vi "CRYO_MASTER_FULL_RUN2.vi"() -> ()   [LabVIEW 2017] (continued)
          }
          frame #47 {
            n631 = Search 1D Array(1D array=w1178, element=T14."TTH4" ("SensorLocations")) -> (index of element=w1175:i32)  [unwired: 1 in]
            n632 = Index Array(array=w1176, index=w1175) -> (element=→"TTH4":dbl)
          }
          frame #48 {
            n633 = Search 1D Array(1D array=w1183, element="SensorLocation 1") -> (index of element=w1180:i32)  [unwired: 1 in]
            n634 = Index Array(array=w1181, index=w1180) -> (element=→"Temperature 1":dbl)
          }
          frame #49 {
            n635 = Search 1D Array(1D array=w1188, element="SensorLocation 2") -> (index of element=w1185:i32)  [unwired: 1 in]
            n636 = Index Array(array=w1186, index=w1185) -> (element=→"Temperature 2":dbl)
          }
        }
      }
      frame #1 {
        n637 = stacked-sequence {
          tunnel: w1190 -> [w1195 w1200 w1205 w1210 w1215 w1220 w1225 w1230 w1235 w1240 w1245 w1250 w1255 w1260 w1265 w1270 w1275 w1280 w1285]
          tunnel: w1189 -> [w1192 w1198 w1204 w1209 w1214 w1218 w1223 w1228 w1233 w1238 w1243 w1248 w1252 w1257 w1262 w1267 w1272 w1277 w1282]
          frame #0 {
            n638 = Search 1D Array(1D array=w1195, element="Insulation vacuum") -> (index of element=w1193:i32)  [unwired: 1 in]
            n639 = Index Array(array=w1192, index=w1193) -> (element=→"P_ins" →"P (insulation)":dbl)
          }
          frame #1 {
            n640 = Search 1D Array(1D array=w1200, element="4K reservoir pressure") -> (index of element=w1197:i32)  [unwired: 1 in]
            n641 = Index Array(array=w1198, index=w1197) -> (element=→"P_4Kres" →"P (4K reservoir)":dbl)
          }
          frame #2 {
            n642 = Search 1D Array(1D array=w1205, element="3He inlet pressure") -> (index of element=w1203:i32)  [unwired: 1 in]
            n643 = Index Array(array=w1204, index=w1203) -> (element=→"P_3HeIN" →"P (3He IN)":dbl)
          }
          frame #3 {
            n644 = Search 1D Array(1D array=w1210, element="Shield return press.") -> (index of element=w1208:i32)  [unwired: 1 in]
            n645 = Index Array(array=w1209, index=w1208) -> (element=→"P_SldRTN" →"P (shield return)":dbl)
          }
          frame #4 {
            n646 = Search 1D Array(1D array=w1215, element="3He pot pressure") -> (index of element=w1213:i32)  [unwired: 1 in]
            n647 = Index Array(array=w1214, index=w1213) -> (element=→"P_3Hepot" →"P (3He pot)":dbl)
          }
          frame #5 {
            n648 = Search 1D Array(1D array=w1220, element="1Kpot pressure") -> (index of element=w1217:i32)  [unwired: 1 in]
            n649 = Index Array(array=w1218, index=w1217) -> (element=→"P_1Kpot" →"P (1K pot)":dbl)
          }
          frame #6 {
            n650 = Search 1D Array(1D array=w1225, element="Dewar pressure") -> (index of element=w1222:i32)  [unwired: 1 in]
            n651 = Index Array(array=w1223, index=w1222) -> (element=→"P_Dewar" →"P (Dewar)":dbl)
          }
          frame #7 {
            n652 = Search 1D Array(1D array=w1230, element="HEX7 out pressure") -> (index of element=w1227:i32)  [unwired: 1 in]
            n653 = Index Array(array=w1228, index=w1227) -> (element=→"P_HEX7OUT" →"P (HEX7 out)":dbl)
          }
          frame #8 {
            n654 = Search 1D Array(1D array=w1235, element="Diff pressure HEX4") -> (index of element=w1232:i32)  [unwired: 1 in]
            n655 = Index Array(array=w1233, index=w1232) -> (element=→"DP_HEX4" →"DP HEX4":dbl)
          }
          frame #9 {
            n656 = Search 1D Array(1D array=w1240, element="Diff pressure HEX5") -> (index of element=w1237:i32)  [unwired: 1 in]
            n657 = Index Array(array=w1238, index=w1237) -> (element=→"DP_HEX5" →"DP HEX5":dbl)
          }
          frame #10 {
            n658 = Search 1D Array(1D array=w1245, element="1K pump exhaust flow") -> (index of element=w1242:i32)  [unwired: 1 in]
            n659 = Index Array(array=w1243, index=w1242) -> (element=→"F_1" →"F1 (1K pump exhaust) flow":dbl)
          }
          frame #11 {
            n660 = Search 1D Array(1D array=w1250, element="Shield flow") -> (index of element=w1247:i32)  [unwired: 1 in]
            n661 = Index Array(array=w1248, index=w1247) -> (element=→"F_2" →"F2 (shield flow)":dbl)
          }
          frame #12 {
            n662 = Search 1D Array(1D array=w1255, element="4He return flow from HEX7") -> (index of element=w1253:i32)  [unwired: 1 in]
            n663 = Index Array(array=w1252, index=w1253) -> (element=→"F_3" →"F3 (4He rtn flw via HEX7)":dbl)
          }
          frame #13 {
            n664 = Search 1D Array(1D array=w1260, element="3He incoming flow into HEX7") -> (index of element=w1258:i32)  [unwired: 1 in]
            n665 = Index Array(array=w1257, index=w1258) -> (element=→"F_4" →"F4 (3He in to HEX7)":dbl)
          }
          frame #14 {
            n666 = Search 1D Array(1D array=w1265, element="3He pump exhaust flow") -> (index of element=w1263:i32)  [unwired: 1 in]
            n667 = Index Array(array=w1262, index=w1263) -> (element=→"F_5" →"F5 (3He pump ex.)":dbl)
          }
          frame #15 {
            n668 = Search 1D Array(1D array=w1270, element="4K reservoir level") -> (index of element=w1268:i32)  [unwired: 1 in]
            n669 = Index Array(array=w1267, index=w1268) -> (element=→"L3" →"He level (4K)":dbl)
          }
          frame #16 {
            n670 = Search 1D Array(1D array=w1275, element="1K pot level") -> (index of element=w1273:i32)  [unwired: 1 in]
            n671 = Index Array(array=w1272, index=w1273) -> (element=→"L(1K) (a1)" →"He level (1K)":dbl)
          }
          frame #17 {
            n672 = Search 1D Array(1D array=w1280, element="1K pot (b)") -> (index of element=w1278:i32)  [unwired: 1 in]
            n673 = Index Array(array=w1277, index=w1278) -> (element=→"1K pot(b1)" →"He level (1K) b":dbl)
          }
          frame #18 {
            n674 = Search 1D Array(1D array=w1285, element="3He pot") -> (index of element=w1283:i32)  [unwired: 1 in]
            n675 = Index Array(array=w1282, index=w1283) -> (element=→"3He pot level" →"He level (3He)":dbl)
          }
        }
      }
    }
    n676 = case shown="False" w830 {
      tunnel: [w1951 w1966] -> w900
      tunnel: [w1946 w1965] -> w917
      tunnel: [w1949 w1964] -> w901
      tunnel: w837 -> [w1950 _]
      tunnel: w916 -> [w1940 w1959]
      tunnel: w915 -> [w1941 w1958]
      tunnel: w862 -> [_ w1957]
      tunnel: [w1938 timestamp[] [] ("TimeArray")] -> w914
      tunnel: [w1937 dbl[][] [] ("DataArray")] -> w913
      frame False {
        w1944 = 24 ("index")
        n677 = local read "Record interval"() -> (w1935:i64)
        n678 = call-dynamic "LSI218Data_measure.vi"("LSI218Data in"=w1941, "MeasurementIndex"=w1950, "error in (no error)"=w1940, "save every ... measurements"=w1935) -> ("TimeMeasuremeent"=→"Time of Last Measurement (LSI218)":timestamp, "Active?"=w1945:bool[], "LSI218Data out"=w1949:refnum<class "LSI218Data.lvclass">, "LastMeasurementConfig"=→"LastMeasurementConfig (218)":T17, "LastData"=w1939:dbl[], "Status"=w1946:u16, "TimeArray"=w1938:timestamp[], "DataArray"=w1937:dbl[][], "error out"=w1951:errorcluster)  [unwired: 3 in]
        "LastData (LSI218)" <- w1939
        n679 = Split 1D Array(array=w1945, index=w1944) -> (first subarray=→"Active?\n (1)":bool[], second subarray=→"Active?\n(2)":bool[])
        n680 = Split 1D Array(array=w1939, index=w1944) -> (first subarray=→"Last Data \nLSI218 (1)":dbl[], second subarray=→"Last Data \nLSI218 (2)":dbl[])
      }
      frame True {
        n681 = local read "RUN Identifier"() -> (w1953:string)
        n682 = call-dynamic "LSI218Data_initialize.vi"("LSI218Settings(A-F)"="LSI218Settings(A-F)", "FileFormat"="FileFormat (218)", "base path"=w1957, "error in (no error)"=w1959, "InstName"="InstName (LSI218)", "RunIdentifier"=w1953, "LSI218Data in"=w1958) -> ("error out"=w1966:errorcluster, "Status"=w1965:T7, "AllLabels"=w1956:string[], "LSI218Data out"=w1964:refnum<class "LSI218Data.lvclass">)  [unwired: 1 in]
        n683 = Split 1D Array(array=w1956, index=24) -> (first subarray=→"Labels LSI218 (1)":string[], second subarray=→"Labels LSI218 (2)":string[])
      }
    }
    "LSI218 Status" <- w917
    "error out (LSI218)" <- w900
    n684 = case shown="True" w830 {
      tunnel: [w1846 w1858] -> w887
      tunnel: [w1836 w1857] -> w895
      tunnel: [w1845 w1856] -> w888
      tunnel: [w1844 timestamp[] [] ("TimeArray")] -> w856
      tunnel: [w1843 dbl[][] [] ("DataArray")] -> w854
      tunnel: w897 -> [w1842 w1853]
      tunnel: w896 -> [w1841 w1852]
      tunnel: w837 -> [w1837 _]
      tunnel: w862 -> [_ w1848]
      frame False {
        n685 = local read "Record interval"() -> (w1834:i64)
        n686 = call-dynamic "LSI336Data_measure.vi"("LSI336Data in"=w1842, "MeasurementIndex"=w1837, "error in (no error)"=w1841, "save every ... measurements"=w1834) -> ("Active?"=→"Active?\n(LSI336)":bool[], "TimeMeasuremeent"=→"Time of Last Measurement (LSI336)":timestamp, "LSI336Data out"=w1845:refnum<class "LSI336Data.lvclass">, "LastData"=→"Last Data \nLSI336":dbl[], "LastMeasurementConfig"=→"LastMeasurementConfig (336)":T17, "DataArray"=w1843:dbl[][], "Status"=w1836:u16, "TimeArray"=w1844:timestamp[], "error out"=w1846:errorcluster)  [unwired: 3 in]
      }
      frame True {
        n687 = local read "RUN Identifier"() -> (w1847:string)
        n688 = call-dynamic "LSI336Data_initialize.vi"("LSI336Data in"=w1853, "RunIdentifier"=w1847, "InstName"="InstName (LSI336)", "FileFormat"="FileFormat (336)", "LSI336Settings(X, Y)"="LSI336Settings(X,Y)", "error in (no error)"=w1852, "base path"=w1848) -> ("LSI336Data out"=w1856:refnum<class "LSI336Data.lvclass">, "Status"=w1857:T7, "AllLabels"=→"Labels LSI336":string[], "error out"=w1858:errorcluster)  [unwired: 5 in]
      }
    }
    "LSI336 Status" <- w895
    "error out (LSI336)" <- w887
    "TimeArray (LSI336)" <- w856
    "DataArray (336)" <- w854
    n689 = local read "Last Data \n(USB6210)"() -> (w840:dbl[])
    n690 = local read "Last Data \n(USB6218)"() -> (w841:dbl[])
    n691 = local read "All Labels (USB6210)"() -> (w843:string[])
    n692 = local read "All Labels (USB6218)"() -> (w842:string[])
    n693 = flat-sequence {
      tunnel: w923 -> [w1425]
      tunnel: [w1420] -> w911
      tunnel: [w1418] -> w909
      tunnel: [w1417] -> w906
      tunnel: [w1416] -> w904
      tunnel: w875 -> [w1411]
      frame #0 {
        w1419 = T25 [] ("appended array")
        n694 = Unbundle By Name(w1411) -> ("TimeArray"=w1428:timestamp[], "DataArrayConv"=w1423:dbl[][], "LDArray"=w1422:dbl[])
        n695 = Unbundle By Name(w1425) -> ("ReadLeakDet?"=w1424:bool, "LabelLD"=w1427:string, "Labels"=w1421:string[])  [unwired: 1 out]
        n696 = case shown="True" w1424 {
          tunnel: w1427 -> [_ w1436]
          tunnel: w1423 -> [w1430 w1435]
          tunnel: w1422 -> [_ w1434]
          tunnel: [w1430 w1433] -> w1410
          tunnel: w1421 -> [w1429 w1432]
          tunnel: [w1429 w1431] -> w1413
          frame False {
          }
          frame True {
            n697 = Build Array (concatenate)(w1435, w1434) -> (w1433:dbl[][])
            n698 = Build Array (concatenate)(w1432, w1436) -> (w1431:string[])
          }
        }
        "All Labels (USB6210)" <- w1413
        "DataArrayConv (USB6210)" <- w1410
        n699 = control-ref of="Plot selecter (USB6210)\n    1      2     3     4"() -> (w1412:refnum<vi>)
        n700 = local read "Plot selecter (USB6210)\n    1      2     3     4"() -> (w1415:bool[][])
        n701 = Array Size(array=w1413) -> (size(s)=w1426:i32)
        n702 = Array Size(array=w1413) -> (size(s)=w1414:i32)
        n703 = Array Size(array=w1410) -> (size(s)=→"Data Array sizes (6210)":i32[])
        n704 = property on="Property Node" class="Arr (strict)"(reference=w1412, "Number of Rows"=w1414) -> ()  [unwired: 1 in, 2 out]
        n705 = for {
          N: w1426 -> [_]
          tunnel: w1410 -> [w1457]
          tunnel: w1428 -> [w1458]
          shift-right: [w1453] -> w1418
          shift-left: w1419 -> [w1456]
          shift-right: [w1451] -> w1416
          shift-left: w1419 -> [w1454]
          shift-right: [w1452] -> w1420
          shift-left: w1419 -> [w1450]
          shift-right: [w1449] -> w1417
          shift-left: w1419 -> [w1448]
          tunnel: w1415 -> [w1447]
          i -> [w1442]
          n706 = Index Array(array=w1457, index (col)=w1442) -> (element=w1437:dbl[])  [unwired: 1 in]
          n707 = Index Array(array=w1447, index (row) #1=w1442, index (col) #1=0 ("index (row)"), index (row) #2=w1442, index (col) #2=1 ("index (row)"), index (row) #3=w1442, index (col) #3=2 ("index (row)"), index (row) #4=w1442, index (col) #4=3 ("index (row)")) -> (element #1=w1441:bool, element #2=w1440:bool, element #3=w1439:bool, element #4=w1438:bool)
          n708 = Bundle("TimeArray"=w1458, "DataArrayConv"=w1437) -> (w1455:T29)  [unwired: 1 in]
          n709 = stacked-sequence {
            tunnel: w1441 -> [w1462 _ _ _]
            tunnel: w1456 -> [_ w1470 _ _]
            tunnel: w1439 -> [_ _ w1478 _]
            tunnel: w1455 -> [w1459 w1468 w1477 w1483]
            tunnel: w1438 -> [_ _ _ w1486]
            tunnel: w1454 -> [_ _ _ w1485]
            tunnel: [_ _ _ w1484] -> w1451
            tunnel: [_ w1469 _ _] -> w1453
            tunnel: [w1461 _ _ _] -> w1452
            tunnel: w1450 -> [w1460 _ _ _]
            tunnel: [_ _ w1476 _] -> w1449
            tunnel: w1448 -> [_ _ w1475 _]
            tunnel: w1440 -> [_ w1467 _ _]
            frame #0 {
              n710 = case shown="True" w1462 {
                tunnel: [w1463 w1466] -> w1461
                tunnel: w1459 -> [_ w1465]
                tunnel: w1460 -> [w1463 w1464]
                frame False {
                }
                frame True {
                  n711 = Build Array (concatenate)(w1464, w1465) -> (w1466:T25)
                }
              }
            }
            frame #1 {
              n712 = case shown="True" w1467 {
                tunnel: w1470 -> [w1471 w1474]
                tunnel: [w1471 w1473] -> w1469
                tunnel: w1468 -> [_ w1472]
                frame False {
                }
                frame True {
                  n713 = Build Array (concatenate)(w1474, w1472) -> (w1473:T25)
                }
              }
            }
            frame #2 {
              n714 = case shown="True" w1478 {
                tunnel: [w1479 w1482] -> w1476
                tunnel: w1477 -> [_ w1481]
                tunnel: w1475 -> [w1479 w1480]
                frame False {
                }
                frame True {
                  n715 = Build Array (concatenate)(w1480, w1481) -> (w1482:T25)
                }
              }
            }
            frame #3 {
              n716 = case shown="True" w1486 {
                tunnel: [w1487 w1490] -> w1484
                tunnel: w1483 -> [_ w1489]
                tunnel: w1485 -> [w1487 w1488]
                frame False {
                }
                frame True {
                  n717 = Build Array (concatenate)(w1488, w1489) -> (w1490:T25)
                }
              }
            }
          }
        }
      }
    }
    n718 = case shown="True" "Digital Out ON?" {
      tunnel: w830 -> [_ w1547]
      tunnel: w877 -> [w1541 w1546]
      tunnel: [w1541 w1545] -> w876
      tunnel: w875 -> [_ w1544]
      tunnel: w862 -> [_ w1543]
      tunnel: w857 -> [_ w1542]
      frame False {
      }
      frame True {
        n719 = case shown="True" w1547 {
          tunnel: w1546 -> [w1565 w1748]
          tunnel: [w1565 w1761] -> w1545
          tunnel: w1544 -> [w1566 _]
          tunnel: w1543 -> [_ w1740]
          tunnel: w1542 -> [_ _]
          frame False {
            n720 = flat-sequence {
              frame #0 {
              }
            }
            n721 = case shown="\"USB6218AI\"" "AutoFill Source (P)" {
              tunnel: [w1569 w1570] -> w1551
              frame "USB6210", Default {
                n722 = local read "All Labels (USB6210)"() -> (w1569:string[])
              }
              frame "USB6218AI" {
                n723 = local read "All Labels (USB6218)"() -> (w1570:string[])
              }
            }
            n724 = case shown="\"USB6210\", Default" "AutoFill Source (L)" {
              tunnel: [w1567 w1568] -> w1548
              frame "USB6210", Default {
                n725 = local read "All Labels (USB6210)"() -> (w1567:string[])
              }
              frame "USB6218AI" {
                n726 = local read "All Labels (USB6218)"() -> (w1568:string[])
              }
            }
            n727 = Multiply(x="N for sampling", y=i64 2) -> (x*y=w1560:i64)
            n728 = local read "Cycle #"() -> (w1564:u32)
            n729 = Search 1D Array(1D array=w1551, element="Auto Fll Dewar P. label") -> (index of element=→"Target Index (P)":i32)  [unwired: 1 in]
            n730 = Search 1D Array(1D array=w1548, element="Auto Fll He L. label") -> (index of element=→"Target Index (L)":i32)  [unwired: 1 in]
            n731 = Add(x=w1560, y="Mov. Avg Interval") -> (x+y=w1562:i64)
            n732 = Greater?(x=w1564, y=w1562) -> (0:w1558:bool)
            n733 = And(x=w1558, y="Auto Fill ON?") -> (x .and. y?=w1556:bool)
            n734 = case shown="True" w1556 {
              tunnel: w1566 -> [_ w1604]
              tunnel: "Mov. Avg Interval" -> [_ w1590]
              tunnel: w1560 -> [_ w1577]
              tunnel: "N for sampling" -> [_ w1588]
              frame False {
              }
              frame True {
                n735 = local read "AutoFill Source (L)"() -> (w1571:T8)
                n736 = local read "AutoFill Source (P)"() -> (w1572:T8)
                n737 = case shown="\"USB6218AI\"" w1572 {
                  tunnel: [w1608 w1609] -> w1573
                  frame "USB6210", Default {
                    n738 = local read "DataArrayConv (USB6210)"() -> (w1608:dbl[][])
                  }
                  frame "USB6218AI" {
                    n739 = local read "DataArrayConv (USB6218)"() -> (w1609:dbl[][])
                  }
                }
                n740 = case shown="\"USB6210\", Default" w1571 {
                  tunnel: [w1606 w1607] -> w1575
                  frame "USB6210", Default {
                    n741 = local read "DataArrayConv (USB6210)"() -> (w1606:dbl[][])
                  }
                  frame "USB6218AI" {
                    n742 = local read "DataArrayConv (USB6218)"() -> (w1607:dbl[][])
                  }
                }
                n743 = local read "Pstd"() -> (→"Pstd history":dbl)
                n744 = local read "Lstd"() -> (→"Lstd history":dbl)
                n745 = local read "Target Index (L)"() -> (w1576:i32)
                n746 = local read "Pav (Pa)"() -> (→"Pav history":dbl)
                n747 = local read "Lav (%)"() -> (→"Lav history":dbl)
                n748 = Index Array(array=w1575, index (col)=w1576) -> (element=w1574:dbl[])  [unwired: 1 in]
                n749 = local read "Target Index (P)"() -> (w1605:i32)
                n750 = Unbundle By Name(w1604) -> ("TimeArray"=w1603:timestamp[])
                n751 = Index Array(array=w1573, index (col)=w1605) -> (element=w1592:dbl[])  [unwired: 1 in]
                n752 = Delete From Array(array=w1592, length=w1577) -> (deleted portion=w1600:dbl[])  [unwired: 1 in, 1 out]
                n753 = Delete From Array(array=w1574, length=w1577) -> (deleted portion=w1587:dbl[])  [unwired: 1 in, 1 out]
                n754 = call "MovingAverage.vi"("Moving Average interval"=w1590, "Input Array"=w1574) -> ("M.A. Array"=w1589:dbl[])  [unwired: 9 in]
                n755 = call "MovingAverage.vi"("Moving Average interval"=w1590, "Input Array"=w1592) -> ("M.A. Array"=w1591:dbl[])  [unwired: 9 in]
                n756 = Delete From Array(array=w1591, length=w1577) -> (deleted portion=w1601:dbl[])  [unwired: 1 in, 1 out]
                n757 = Delete From Array(array=w1591, length=w1577) -> (deleted portion=w1597:dbl[])  [unwired: 1 in, 1 out]
                "Last N M.A. Pressures" <- w1597
                n758 = Delete From Array(array=w1589, length=w1577) -> (deleted portion=w1582:dbl[])  [unwired: 1 in, 1 out]
                "Last N M.A. Levels" <- w1582
                n759 = Delete From Array(array=w1603, length=w1577) -> (deleted portion=w1584:timestamp[])  [unwired: 1 in, 1 out]
                n760 = Bundle("TimeArray"=w1584, "DataArrayConv (USB6218)"=w1600) -> (w1599:T30)  [unwired: 1 in]
                n761 = Bundle("TimeArray"=w1584, "M.A. Array"=w1601) -> (w1602:T31)  [unwired: 1 in]
                n762 = Bundle("TimeArray"=w1584, "DataArrayConv (USB6218)"=w1587) -> (w1586:T30)  [unwired: 1 in]
                n763 = Bundle("TimeArray"=w1584, "M.A. Array"=w1582) -> (w1583:T31)  [unwired: 1 in]
                n764 = Array Size(array=w1597) -> (size(s)=w1596:i32)
                n765 = Greater Or Equal?(x=w1596, y=w1588) -> (x >= y?=w1595:bool)
                n766 = Build Array(w1599, w1602) -> (→"Dewar Pressure":T32)
                n767 = Build Array(w1586, w1583) -> (→"He Level":T32)
                n768 = case shown="True" w1595 {
                  tunnel: [w1713 w1718] -> w1581
                  tunnel: w1597 -> [_ w1719]
                  tunnel: w1582 -> [_ w1716]
                  tunnel: [w1713 w1714] -> w1580
                  frame False {
                    w1713 = nan ("mean")
                  }
                  frame True {
                    n769 = call <vilib>:"Std Deviation and Variance.vi"("X"=w1719) -> ("mean"=w1718:dbl, "standard deviation"=w1717:dbl)  [unwired: 1 in, 1 out]
                    n770 = call <vilib>:"Std Deviation and Variance.vi"("X"=w1716) -> ("mean"=w1714:dbl, "standard deviation"=w1715:dbl)  [unwired: 1 in, 1 out]
                    n771 = local write "Pstd"(w1717) -> ()
                    n772 = local write "Lstd"(w1715) -> ()
                    n773 = local write "Pav (Pa)"(w1718) -> ()
                    n774 = local write "Lav (%)"(w1714) -> ()
                  }
                }
                n775 = flat-sequence {
                  tunnel: w1581 -> [w1610]
                  tunnel: w1580 -> [w1611]
                  frame #0 {
                    n776 = flat-sequence {
                      tunnel: w1611 -> [w1613]
                      tunnel: w1610 -> [w1612]
                      tunnel: w1610 -> [w1681]
                      frame #0 {
                        n777 = stacked-sequence {
                          tunnel: w1613 -> [w1620 w1624 _ _ _ _]
                          tunnel: w1612 -> [_ _ w1638 w1647 w1656 w1665]
                          frame #0 {
                            n778 = local read "L_low (%)"() -> (w1619:dbl)
                            n779 = local read "Fill state"() -> (w1617:bool)
                            n780 = Less?(x=w1620, y=w1619) -> (x < y?=w1616:bool)
                            n781 = Equal?(x=w1617, y=FALSE) -> (x = y?=w1615:bool)
                            n782 = And(x=w1616, y=w1615) -> (x .and. y?=w1614:bool)
                            n783 = case shown="False" w1614 {
                              frame False {
                              }
                              frame True {
                                w1622 = TRUE ("Value (Signaling)")
                                n784 = property on="Fill state" class="Bool (strict)"("Val(Sgnl)"=w1622) -> ()  [unwired: 2 in, 2 out]
                                n785 = Not(x=w1622) -> (.not. x?=w1621:bool)
                                n786 = property on="Fill (false)" class="Bool (strict)"("Val(Sgnl)"=w1621) -> ()  [unwired: 2 in, 2 out]
                              }
                            }
                          }
                          frame #1 {
                            n787 = local read "L_high (%)"() -> (w1625:dbl)
                            n788 = local read "Fill state"() -> (w1628:bool)
                            n789 = Greater?(x=w1624, y=w1625) -> (0:w1623:bool)
                            n790 = Equal?(x=w1628, y=TRUE) -> (x = y?=w1627:bool)
                            n791 = And(x=w1623, y=w1627) -> (x .and. y?=w1626:bool)
                            n792 = case shown="True" w1626 {
                              frame False {
                              }
                              frame True {
                                w1630 = FALSE ("Value (Signaling)")
                                n793 = property on="Fill state" class="Bool (strict)"("Val(Sgnl)"=w1630) -> ()  [unwired: 2 in, 2 out]
                                n794 = Not(x=w1630) -> (.not. x?=w1631:bool)
                                n795 = property on="Fill (false)" class="Bool (strict)"("Val(Sgnl)"=w1631) -> ()  [unwired: 2 in, 2 out]
                              }
                            }
                          }
                          frame #2 {
                            n796 = local read "P_1_low (Pa)"() -> (w1637:dbl)
                            n797 = property on="state 1" class="Bool (strict)"() -> ("Value"=w1635:bool)  [unwired: 2 in, 2 out]
                            n798 = Less?(x=w1638, y=w1637) -> (x < y?=w1634:bool)
                            n799 = Equal?(x=w1635, y=FALSE) -> (x = y?=w1633:bool)
                            n800 = And(x=w1633, y=w1634) -> (x .and. y?=w1632:bool)
                            n801 = case shown="True" w1632 {
                              frame False {
                              }
                              frame True {
                                w1640 = TRUE ("Value (Signaling)")
                                n802 = property on="state 1" class="Bool (strict)"("Val(Sgnl)"=w1640) -> ()  [unwired: 2 in, 2 out]
                                n803 = Not(x=w1640) -> (.not. x?=w1639:bool)
                                n804 = property on="state 1 (false)" class="Bool (strict)"("Val(Sgnl)"=w1639) -> ()  [unwired: 2 in, 2 out]
                              }
                            }
                          }
                          frame #3 {
                            n805 = local read "P_1_high (Pa)"() -> (w1646:dbl)
                            n806 = property on="state 1" class="Bool (strict)"() -> ("Value"=w1644:bool)  [unwired: 2 in, 2 out]
                            n807 = Greater?(x=w1647, y=w1646) -> (0:w1643:bool)
                            n808 = Equal?(x=w1644, y=TRUE) -> (x = y?=w1642:bool)
                            n809 = And(x=w1642, y=w1643) -> (x .and. y?=w1641:bool)
                            n810 = case shown="True" w1641 {
                              frame False {
                              }
                              frame True {
                                w1649 = FALSE ("Value (Signaling)")
                                n811 = property on="state 1" class="Bool (strict)"("Val(Sgnl)"=w1649) -> ()  [unwired: 2 in, 2 out]
                                n812 = Not(x=w1649) -> (.not. x?=w1648:bool)
                                n813 = property on="state 1 (false)" class="Bool (strict)"("Val(Sgnl)"=w1648) -> ()  [unwired: 2 in, 2 out]
                              }
                            }
                          }
                          frame #4 {
                            n814 = local read "P_2_low (Pa)"() -> (w1655:dbl)
                            n815 = property on="state 2" class="Bool (strict)"() -> ("Value"=w1650:bool)  [unwired: 2 in, 2 out]
                            n816 = Less?(x=w1656, y=w1655) -> (x < y?=w1653:bool)
                            n817 = Equal?(x=w1650, y=FALSE) -> (x = y?=w1652:bool)
                            n818 = And(x=w1652, y=w1653) -> (x .and. y?=w1651:bool)
                            n819 = case shown="True" w1651 {
                              frame False {
                              }
                              frame True {
                                w1657 = TRUE ("Value (Signaling)")
                                n820 = property on="state 2" class="Bool (strict)"("Val(Sgnl)"=w1657) -> ()  [unwired: 2 in, 2 out]
                                n821 = Not(x=w1657) -> (.not. x?=w1658:bool)
                                n822 = property on="state 2 (false)" class="Bool (strict)"("Val(Sgnl)"=w1658) -> ()  [unwired: 2 in, 2 out]
                              }
                            }
                          }
                          frame #5 {
                            n823 = local read "P_2_high (Pa)"() -> (w1664:dbl)
                            n824 = property on="state 2" class="Bool (strict)"() -> ("Value"=w1659:bool)  [unwired: 2 in, 2 out]
                            n825 = Greater?(x=w1665, y=w1664) -> (0:w1662:bool)
                            n826 = Equal?(x=w1659, y=TRUE) -> (x = y?=w1661:bool)
                            n827 = And(x=w1661, y=w1662) -> (x .and. y?=w1660:bool)
                            n828 = case shown="True" w1660 {
                              frame False {
                              }
                              frame True {
                                w1666 = FALSE ("Value (Signaling)")
                                n829 = property on="state 2" class="Bool (strict)"("Val(Sgnl)"=w1666) -> ()  [unwired: 2 in, 2 out]
                                n830 = Not(x=w1666) -> (.not. x?=w1667:bool)
                                n831 = property on="state 2 (false)" class="Bool (strict)"("Val(Sgnl)"=w1667) -> ()  [unwired: 2 in, 2 out]
                              }
                            }
                          }
                        }
                      }
                      frame #1 {
                        n832 = property on="Fill state" class="Bool (strict)"() -> ("Value"=w1668:bool)  [unwired: 2 in, 2 out]
                        n833 = case shown="True" w1668 {
                          frame False {
                            n834 = property on="V1 (N.O.)" class="Bool (strict)"("Val(Sgnl)"=TRUE ("V1 (N.O.)")) -> ()  [unwired: 2 in, 2 out]
                            n835 = property on="V2 (N.C.)" class="Bool (strict)"("Val(Sgnl)"=FALSE ("Value (Signaling)")) -> ()  [unwired: 2 in, 2 out]
                          }
                          frame True {
                            n836 = property on="state 1" class="Bool (strict)"() -> ("Value"=w1672:bool)  [unwired: 2 in, 2 out]
                            n837 = property on="state 2" class="Bool (strict)"() -> ("Value"=w1671:bool)  [unwired: 2 in, 2 out]
                            n838 = case shown="True" w1672 {
                              frame False {
                                n839 = property on="V1 (N.O.)" class="Bool (strict)"("Val(Sgnl)"=TRUE ("Value (Signaling)")) -> ()  [unwired: 2 in, 2 out]
                                n840 = local write "Status V1 CTRL"(enum16{"Pressurize", "Release"}."Release" ("Status V1 CTRL")) -> ()
                              }
                              frame True {
                                n841 = property on="V1 (N.O.)" class="Bool (strict)"("Val(Sgnl)"=FALSE ("V1 (N.O.)")) -> ()  [unwired: 2 in, 2 out]
                                n842 = local write "Status V1 CTRL"(enum16{"Pressurize", "Release"}."Pressurize" ("Status V1 CTRL")) -> ()
                              }
                            }
                            n843 = case shown="True" w1671 {
                              frame False {
                                n844 = property on="V2 (N.C.)" class="Bool (strict)"("Val(Sgnl)"=FALSE ("Value (Signaling)")) -> ()  [unwired: 2 in, 2 out]
                                n845 = local write "Status V2 CTRL"(enum16{"Pressurize", "Release"}."Release" ("Status V2 CTRL")) -> ()
                              }
                              frame True {
                                n846 = property on="V2 (N.C.)" class="Bool (strict)"("Val(Sgnl)"=TRUE ("Value (Signaling)")) -> ()  [unwired: 2 in, 2 out]
                                n847 = local write "Status V2 CTRL"(enum16{"Pressurize", "Release"}."Pressurize" ("Status V2 CTRL")) -> ()
                              }
                            }
                          }
                        }
                      }
                      frame #2 {
                        n848 = Greater?(x=w1681, y="P_safelimit_high (Pa)") -> (0:w1683:bool)
                        n849 = Less?(x=w1681, y="P_safelimit_low (Pa)") -> (x < y?=w1685:bool)
                        n850 = Or(x=w1683, y=w1685) -> (x .or. y?=w1686:bool)
                        n851 = case shown="False" w1686 {
                          frame False {
                          }
                          frame True {
                            w1687 = FALSE ("Value (Signaling)")
                            w1689 = FALSE ("Value (Signaling)")
                            n852 = property on="V2 (N.C.)" class="Bool (strict)"("Val(Sgnl)"=FALSE ("V1 (N.O.)")) -> ()  [unwired: 2 in, 2 out]
                            n853 = property on="state 1" class="Bool (strict)"("Val(Sgnl)"=w1687) -> ()  [unwired: 2 in, 2 out]
                            n854 = property on="V1 (N.O.)" class="Bool (strict)"("Val(Sgnl)"=TRUE ("V1 (N.O.)")) -> ()  [unwired: 2 in, 2 out]
                            n855 = property on="state 2" class="Bool (strict)"("Val(Sgnl)"=w1689) -> ()  [unwired: 2 in, 2 out]
                            n856 = Not(x=w1687) -> (.not. x?=w1688:bool)
                            n857 = Not(x=w1689) -> (.not. x?=w1690:bool)
                            n858 = property on="state 1 (false)" class="Bool (strict)"("Val(Sgnl)"=w1688) -> ()  [unwired: 2 in, 2 out]
                            n859 = property on="state 2 (false)" class="Bool (strict)"("Val(Sgnl)"=w1690) -> ()  [unwired: 2 in, 2 out]
                          }
                        }
                      }
                    }
                  }
                  frame #1 {
                    n860 = property on="V2 (N.C.)" class="Bool (strict)"() -> ("Value"=w1700:bool)  [unwired: 2 in, 2 out]
                    n861 = property on="V1 (N.O.)" class="Bool (strict)"() -> ("Value"=w1711:bool)  [unwired: 2 in, 2 out]
                    n862 = local read "P_1_high (Pa)"() -> (w1705:dbl)
                    n863 = local read "P_2_high (Pa)"() -> (w1703:dbl)
                    n864 = local read "P_1_low (Pa)"() -> (w1706:dbl)
                    n865 = local read "P_2_low (Pa)"() -> (w1704:dbl)
                    n866 = local read "L_high (%)"() -> (w1701:dbl)
                    n867 = local read "L_low (%)"() -> (w1702:dbl)
                    n868 = local read "Pav (Pa)"() -> (w1694:dbl)
                    n869 = local read "Lav (%)"() -> (w1693:dbl)
                    n870 = Boolean To (0,1)(Boolean=w1700) -> (0, 1=w1699:i16)
                    n871 = Boolean To (0,1)(Boolean=w1711) -> (0, 1=w1712:i16)
                    n872 = local read "File Refn DewarCTRL"() -> (w1707:refnum<file>)
                    n873 = local read "Cycle #"() -> (w1710:u32)
                    n874 = Build Array(w1694, w1693, w1706, w1705, w1704, w1703, w1702, w1701, w1712, w1699) -> (w1698:dbl[])
                    n875 = Get Date/Time In Seconds() -> (seconds since 1Jan1904=w1708:timestamp)
                    n876 = call "FileWrite.vi"("DataArray"=w1698, "Time Stamp"=w1708, "Error In"=errorcluster {"status"=FALSE, "code"=0, "source"=""}, "FileFormat"=string[] ["%4.5e", "%4.2f", "%4.4e", "%4.4e", "%4.4e", "%4.4e", "%4.4e", "%d", "%d"] ("Array"), "Index"=w1710, "refnum in"=w1707) -> ("Error Out"=→"Error Out (Dewar CTRL":errorcluster, "Byte Stream File Refnum"=w1697:refnum<file>)  [unwired: 4 in]
                    n877 = local write "File Refn DewarCTRL"(w1697) -> ()
                  }
                }
              }
            }
          }
          frame True {
            w1758 = "_"
            w1721 = FALSE ("auto cleanup")
            w1723 = 1 items=["one channel for each line", "one channel for all lines"] ("line grouping")
            n878 = flat-sequence {
              frame #0 {
                w1775 = FALSE ("V1 (N.O.)")
                n879 = local write "V1 (N.O.)"(TRUE ("V1 (N.O.)")) -> ()
                n880 = local write "V2 (N.C.)"(FALSE ("V1 (N.O.)")) -> ()
                n881 = local write "state 2"(w1775) -> ()
                n882 = local write "state 1"(w1775) -> ()
                n883 = local write "Fill state"(w1775) -> ()
                n884 = Not(x=w1775) -> (.not. x?=w1777:bool)
                n885 = Not(x=w1775) -> (.not. x?=w1776:bool)
                n886 = local write "state 1 (false)"(w1776) -> ()
                n887 = local write "state 2 (false)"(w1776) -> ()
                n888 = local write "Fill (false)"(w1777) -> ()
              }
            }
            n889 = Get Date/Time In Seconds() -> (seconds since 1Jan1904=w1772:timestamp)
            n890 = call "LV_UNIXTIME.vi"("current time"=w1772) -> ("date/time string"=w1753:string)  [unwired: 9 in, 1 out]
            n891 = local read "RUN Identifier"() -> (w1720:string)
            n892 = Concatenate Strings(w1753, "_DO" ("new task name")) -> (w1769:string)
            n893 = Concatenate Strings(w1720, w1758, w1753, w1758) -> (w1739:string)
            n894 = Concatenate Strings(w1739, "DEWAR.csv" ("string")) -> (w1738:string)
            n895 = Concatenate Strings(w1739, "USB_DOUT.csv" ("string")) -> (w1742:string)
            n896 = Build Path(base path=w1740, name or relative path=w1738) -> (appended path=w1737:path)
            n897 = Build Path(base path=w1740, name or relative path=w1742) -> (appended path=w1757:path)
            n898 = Open/Create/Replace File(file path (use dialog)=w1757, error in=w1748, operation (0:open)=T24."open or create") -> (refnum out=w1755:refnum<file>, error out=w1747:errorcluster)  [unwired: 3 in, 1 out]
            n899 = call "FileIntialize.vi"("Error In"=w1747, "Labels"="DOUT Labels", "refnum in"=w1755) -> ("Error Out"=w1734:errorcluster, "File Refnum"=→"File Refn USB DO":refnum<file>)  [unwired: 7 in]
            n900 = Open/Create/Replace File(file path (use dialog)=w1737, error in=w1734, operation (0:open)=T24."open or create") -> (refnum out=w1745:refnum<file>, error out=w1746:errorcluster)  [unwired: 3 in, 1 out]
            n901 = call "FileIntialize.vi"("Error In"=w1746, "Labels"=string[] ["P_av", "L_av", "P_1_low", "P_1_high", "P_2_low", "P_2_high", "L_low", "L_high", "V1(NO)", "V2(NC)"], "refnum in"=w1745) -> ("Error Out"=w1733:errorcluster, "File Refnum"=→"File Refn DewarCTRL":refnum<file>)  [unwired: 7 in]
            n902 = Index Array(array="DOUT Physical CH", index #1=0 ("index"), index #2=1 ("index"), index #3=2 ("index"), index #4=3 ("index")) -> (element #1=w1751:tag, element #2=w1729:tag, element #3=w1728:tag, element #4=w1722:tag)
            n903 = call <vilib>:"DAQmx Create Task.vi"("new task name"=w1769, "auto cleanup"=FALSE, "error in"=w1733) -> ("task out"=w1770:refnum<k21>, "error out"=w1771:errorcluster)  [unwired: 11 in]
            n904 = call-poly <vilib>:"DAQmx Create Virtual Channel.vi"("task in"=w1770, "lines"=w1751, "line grouping"=w1723, "error in"=w1771) -> ("task out"=w1773:refnum<k21>, "error out"=w1774:errorcluster)  [unwired: 10 in]
            n905 = call-poly <vilib>:"DAQmx Create Virtual Channel.vi"("task in"=w1773, "lines"=w1729, "line grouping"=w1723, "error in"=w1774) -> ("task out"=w1760:refnum<k21>, "error out"=w1759:errorcluster)  [unwired: 10 in]
            n906 = call-poly <vilib>:"DAQmx Create Virtual Channel.vi"("task in"=w1760, "lines"=w1728, "line grouping"=w1723, "error in"=w1759) -> ("task out"=w1727:refnum<k21>, "error out"=w1726:errorcluster)  [unwired: 10 in]
            n907 = call-poly <vilib>:"DAQmx Create Virtual Channel.vi"("task in"=w1727, "lines"=w1722, "line grouping"=w1723, "error in"=w1726) -> ("task out"=w1724:refnum<k21>, "error out"=w1725:errorcluster)  [unwired: 10 in]
            n908 = call <vilib>:"DAQmx Start Task.vi"("task/channels in"=w1724, "error in"=w1725) -> ("task out"=w1764:refnum<k21>, "error out"=w1762:errorcluster)  [unwired: 12 in]
            n909 = Build Array(w1721, w1721, w1721, w1721) -> (w1765:bool[])
            n910 = call <vilib>:"DAQmx Write (Digital 1D Bool NChan 1Samp 1Line).vi"("task/channels in"=w1764, "data"=w1765, "timeout"=10.0, "error in"=w1762) -> ("task out"=→"DOUT task out":refnum<k21>, "error out"=w1761:errorcluster)  [unwired: 9 in, 1 out]
          }
        }
      }
    }
    "error out (USB6210/6218 DOUT)" <- w876
    n911 = flat-sequence {
      tunnel: w871 -> [w1344]
      tunnel: [w1339] -> w870
      tunnel: [w1337] -> w869
      tunnel: [w1336] -> w868
      tunnel: [w1335] -> w867
      tunnel: w872 -> [w1331]
      frame #0 {
        w1338 = T25 [] ("appended array")
        n912 = Unbundle By Name(w1331) -> ("TimeArray"=w1327:timestamp[], "DataArrayConv"=w1342:dbl[][], "LDArray"=w1341:dbl[])
        "TimeArray (USB6218)" <- w1327
        n913 = Unbundle By Name(w1344) -> ("ReadLeakDet?"=w1343:bool, "LabelLD"=w1346:string, "Labels"=w1340:string[])  [unwired: 1 out]
        n914 = case shown="True" w1343 {
          tunnel: w1346 -> [_ w1354]
          tunnel: w1342 -> [w1348 w1353]
          tunnel: w1341 -> [_ w1352]
          tunnel: [w1348 w1351] -> w1329
          tunnel: w1340 -> [w1347 w1350]
          tunnel: [w1347 w1349] -> w1332
          frame False {
          }
          frame True {
            n915 = Build Array (concatenate)(w1353, w1352) -> (w1351:dbl[][])
            n916 = Build Array (concatenate)(w1350, w1354) -> (w1349:string[])
          }
        }
        "All Labels (USB6218)" <- w1332
        "DataArrayConv (USB6218)" <- w1329
        n917 = Array Size(array=w1327) -> (size(s)=→"TimeArray size (6218)":i32)
        n918 = local read "Plot selecter (USB6218)\n    1      2     3     4"() -> (w1334:bool[][])
        n919 = control-ref of="Plot selecter (USB6218)\n    1      2     3     4"() -> (w1330:refnum<vi>)
        n920 = Array Size(array=w1332) -> (size(s)=w1333:i32)
        n921 = Array Size(array=w1332) -> (size(s)=w1345:i32)
        n922 = Array Size(array=w1329) -> (size(s)=→"DataArraySize (6218)":i32[])
        n923 = property on="Property Node" class="Arr (strict)"(reference=w1330, "Number of Rows"=w1333) -> ()  [unwired: 1 in, 2 out]
        n924 = for {
          N: w1345 -> [_]
          tunnel: w1329 -> [w1375]
          tunnel: w1327 -> [w1376]
          shift-right: [w1370] -> w1337
          shift-left: w1338 -> [w1373]
          shift-right: [w1368] -> w1335
          shift-left: w1338 -> [w1371]
          shift-right: [w1369] -> w1339
          shift-left: w1338 -> [w1367]
          shift-right: [w1366] -> w1336
          shift-left: w1338 -> [w1365]
          tunnel: w1334 -> [w1364]
          i -> [w1359]
          n925 = Index Array(array=w1375, index (col)=w1359) -> (element=w1374:dbl[])  [unwired: 1 in]
          n926 = Index Array(array=w1364, index (row) #1=w1359, index (col) #1=0 ("index (row)"), index (row) #2=w1359, index (col) #2=1 ("index (row)"), index (row) #3=w1359, index (col) #3=2 ("index (row)"), index (row) #4=w1359, index (col) #4=3 ("index (row)")) -> (element #1=w1358:bool, element #2=w1357:bool, element #3=w1356:bool, element #4=w1355:bool)
          n927 = Bundle("TimeArray"=w1376, "DataArrayConv"=w1374) -> (w1372:T29)  [unwired: 1 in]
          n928 = stacked-sequence {
            tunnel: w1358 -> [w1380 _ _ _]
            tunnel: w1373 -> [_ w1388 _ _]
            tunnel: w1356 -> [_ _ w1396 _]
            tunnel: w1372 -> [w1377 w1386 w1395 w1401]
            tunnel: w1355 -> [_ _ _ w1404]
            tunnel: w1371 -> [_ _ _ w1403]
            tunnel: [_ _ _ w1402] -> w1368
            tunnel: [_ w1387 _ _] -> w1370
            tunnel: [w1379 _ _ _] -> w1369
            tunnel: w1367 -> [w1378 _ _ _]
            tunnel: [_ _ w1394 _] -> w1366
            tunnel: w1365 -> [_ _ w1393 _]
            tunnel: w1357 -> [_ w1385 _ _]
            frame #0 {
              n929 = case shown="True" w1380 {
                tunnel: [w1381 w1384] -> w1379
                tunnel: w1377 -> [_ w1383]
                tunnel: w1378 -> [w1381 w1382]
                frame False {
                }
                frame True {
                  n930 = Build Array (concatenate)(w1382, w1383) -> (w1384:T25)
                }
              }
            }
            frame #1 {
              n931 = case shown="True" w1385 {
                tunnel: w1388 -> [w1389 w1392]
                tunnel: [w1389 w1391] -> w1387
                tunnel: w1386 -> [_ w1390]
                frame False {
                }
                frame True {
                  n932 = Build Array (concatenate)(w1392, w1390) -> (w1391:T25)
                }
              }
            }
            frame #2 {
              n933 = case shown="True" w1396 {
                tunnel: [w1397 w1400] -> w1394
                tunnel: w1395 -> [_ w1399]
                tunnel: w1393 -> [w1397 w1398]
                frame False {
                }
                frame True {
                  n934 = Build Array (concatenate)(w1398, w1399) -> (w1400:T25)
                }
              }
            }
            frame #3 {
              n935 = case shown="True" w1404 {
                tunnel: [w1405 w1408] -> w1402
                tunnel: w1401 -> [_ w1407]
                tunnel: w1403 -> [w1405 w1406]
                frame False {
                }
                frame True {
                  n936 = Build Array (concatenate)(w1406, w1407) -> (w1408:T25)
                }
              }
            }
          }
        }
      }
    }
    n937 = Build Array (concatenate)(w840, w841) -> (w838:dbl[])
    n938 = Build Array (concatenate)(w843, w842) -> (w839:string[])
    n939 = local read "Plot selecter LSI218(2)\n    1      2     3     4"() -> (w898:bool[][])
    n940 = local read "Plot selecter LSI218(1)\n    1      2     3     4"() -> (w899:bool[][])
    n941 = for {
      N: 48 -> [_]
      tunnel: w914 -> [w1879]
      tunnel: w913 -> [w1876]
      tunnel: w899 -> [w1860]
      tunnel: w898 -> [w1861]
      shift-right: [w1877] -> w912
      shift-left: w910 -> [w1878]
      shift-right: [w1872] -> w907
      shift-left: w910 -> [w1873]
      shift-right: [w1871] -> w905
      shift-left: w910 -> [w1870]
      shift-right: [w1869] -> w903
      shift-left: w910 -> [w1868]
      i -> [w1866]
      n942 = Index Array(array=w1876, index (col)=w1866) -> (element=w1875:dbl[])  [unwired: 1 in]
      n943 = Less?(x=w1866, y=24) -> (x < y?=w1867:bool)
      n944 = case shown="True" w1867 {
        tunnel: [w1884 w1902] -> w1865
        tunnel: [w1883 w1901] -> w1864
        tunnel: [w1882 w1899] -> w1863
        tunnel: [w1881 w1898] -> w1862
        tunnel: w1860 -> [_ w1897]
        tunnel: w1861 -> [w1891 _]
        tunnel: w1866 -> [w1886 w1894]
        frame False {
          n945 = Subtract(x=w1886, y=24) -> (x-y=w1890:i32)
          n946 = Index Array(array=w1891, index (row) #1=w1890, index (col) #1=0 ("index (row)"), index (row) #2=w1890, index (col) #2=1 ("index (row)"), index (row) #3=w1890, index (col) #3=2 ("index (row)"), index (row) #4=w1890, index (col) #4=3 ("index (row)")) -> (element #1=w1884:bool, element #2=w1883:bool, element #3=w1882:bool, element #4=w1881:bool)
        }
        frame True {
          n947 = Index Array(array=w1897, index (row) #1=w1894, index (col) #1=0 ("index (row)"), index (row) #2=w1894, index (col) #2=1 ("index (row)"), index (row) #3=w1894, index (col) #3=2 ("index (row)"), index (row) #4=w1894, index (col) #4=3 ("index (row)")) -> (element #1=w1902:bool, element #2=w1901:bool, element #3=w1899:bool, element #4=w1898:bool)
        }
      }
      n948 = Bundle("TimeArray"=w1879, "DataArray"=w1875) -> (w1874:T33)  [unwired: 1 in]
      n949 = stacked-sequence {
        tunnel: w1878 -> [w1906 _ _ _]
        tunnel: [w1905 _ _ _] -> w1877
        tunnel: w1874 -> [w1904 w1914 w1922 w1930]
        tunnel: w1873 -> [_ w1913 _ _]
        tunnel: [_ w1912 _ _] -> w1872
        tunnel: [_ _ w1921 _] -> w1871
        tunnel: w1870 -> [_ _ w1920 _]
        tunnel: [_ _ _ w1929] -> w1869
        tunnel: w1868 -> [_ _ _ w1928]
        tunnel: w1865 -> [w1903 _ _ _]
        tunnel: w1864 -> [_ w1911 _ _]
        tunnel: w1863 -> [_ _ w1919 _]
        tunnel: w1862 -> [_ _ _ w1927]
        frame #0 {
          n950 = case shown="False" w1903 {
            tunnel: w1904 -> [_ w1908]
            tunnel: w1906 -> [w1907 w1910]
            tunnel: [w1907 w1909] -> w1905
            frame False {
            }
            frame True {
              n951 = Build Array (concatenate)(w1910, w1908) -> (w1909:T4)
            }
          }
        }
        frame #1 {
          n952 = case shown="True" w1911 {
            tunnel: [w1915 w1918] -> w1912
            tunnel: w1914 -> [_ w1917]
            tunnel: w1913 -> [w1915 w1916]
            frame False {
            }
            frame True {
              n953 = Build Array (concatenate)(w1916, w1917) -> (w1918:T4)
            }
          }
        }
        frame #2 {
          n954 = case shown="True" w1919 {
            tunnel: [w1923 w1926] -> w1921
            tunnel: w1922 -> [_ w1925]
            tunnel: w1920 -> [w1923 w1924]
            frame False {
            }
            frame True {
              n955 = Build Array (concatenate)(w1924, w1925) -> (w1926:T4)
            }
          }
        }
        frame #3 {
          n956 = case shown="True" w1927 {
            tunnel: [w1931 w1934] -> w1929
            tunnel: w1930 -> [_ w1933]
            tunnel: w1928 -> [w1931 w1932]
            frame False {
            }
            frame True {
              n957 = Build Array (concatenate)(w1932, w1933) -> (w1934:T4)
            }
          }
        }
      }
    }
    n958 = local read "Labels LSI336"() -> (w886:string[])
    n959 = Array Size(array=w886) -> (size(s)=w885:i32)
    n960 = local read "Plot selecter LSI336 \n     1      2     3     4"() -> (w894:bool[][])
    n961 = for {
      N: w885 -> [_]
      tunnel: w894 -> [w1792]
      shift-right: [w1786] -> w892
      shift-left: w893 -> [w1801]
      shift-right: [w1782] -> w891
      shift-left: w893 -> [w1799]
      shift-right: [w1783] -> w890
      shift-left: w893 -> [w1798]
      shift-right: [w1781] -> w889
      shift-left: w893 -> [w1797]
      tunnel: w854 -> [w1789]
      tunnel: w856 -> [w1787]
      i -> [w1790]
      n962 = Index Array(array=w1789, index (col)=w1790) -> (element=w1788:dbl[])  [unwired: 1 in]
      n963 = Index Array(array=w1792, index (row) #1=w1790, index (col) #1=0 ("index (row)"), index (row) #2=w1790, index (col) #2=1 ("index (row)"), index (row) #3=w1790, index (col) #3=2 ("index (row)"), index (row) #4=w1790, index (col) #4=3 ("index (row)")) -> (element #1=w1791:bool, element #2=w1785:bool, element #3=w1784:bool, element #4=w1780:bool)
      n964 = Bundle("TimeArray"=w1787, "DataArray"=w1788) -> (w1800:T33)  [unwired: 1 in]
      n965 = stacked-sequence {
        tunnel: w1801 -> [w1805 _ _ _]
        tunnel: [w1804 _ _ _] -> w1786
        tunnel: w1800 -> [w1803 w1813 w1821 w1829]
        tunnel: w1799 -> [_ w1812 _ _]
        tunnel: [_ w1811 _ _] -> w1782
        tunnel: [_ _ w1820 _] -> w1783
        tunnel: w1798 -> [_ _ w1819 _]
        tunnel: [_ _ _ w1828] -> w1781
        tunnel: w1797 -> [_ _ _ w1827]
        tunnel: w1791 -> [w1802 _ _ _]
        tunnel: w1785 -> [_ w1810 _ _]
        tunnel: w1784 -> [_ _ w1818 _]
        tunnel: w1780 -> [_ _ _ w1826]
        frame #0 {
          n966 = case shown="False" w1802 {
            tunnel: w1803 -> [_ w1807]
            tunnel: w1805 -> [w1806 w1809]
            tunnel: [w1806 w1808] -> w1804
            frame False {
            }
            frame True {
              n967 = Build Array (concatenate)(w1809, w1807) -> (w1808:T4)
            }
          }
        }
        frame #1 {
          n968 = case shown="True" w1810 {
            tunnel: [w1814 w1817] -> w1811
            tunnel: w1813 -> [_ w1815]
            tunnel: w1812 -> [w1814 w1816]
            frame False {
            }
            frame True {
              n969 = Build Array (concatenate)(w1816, w1815) -> (w1817:T4)
            }
          }
        }
        frame #2 {
          n970 = case shown="True" w1818 {
            tunnel: [w1822 w1825] -> w1820
            tunnel: w1821 -> [_ w1823]
            tunnel: w1819 -> [w1822 w1824]
            frame False {
            }
            frame True {
              n971 = Build Array (concatenate)(w1824, w1823) -> (w1825:T4)
            }
          }
        }
        frame #3 {
          n972 = case shown="True" w1826 {
            tunnel: [w1830 w1833] -> w1828
            tunnel: w1829 -> [_ w1831]
            tunnel: w1827 -> [w1830 w1832]
            frame False {
            }
            frame True {
              n973 = Build Array (concatenate)(w1832, w1831) -> (w1833:T4)
            }
          }
        }
      }
    }
    n974 = Array Size(array=w856) -> (size(s)=→"TimeArray Size (336)":i32)
    n975 = Array Size(array=w854) -> (size(s)=→"DataArray size (336)":i32[])
    n976 = Build Array (concatenate)(w906, w905, w890, w868) -> (→"Graph 3":T25)
    n977 = Build Array (concatenate)(w911, w912, w892, w870) -> (→"Graph 1":T25)
    n978 = Build Array (concatenate)(w909, w907, w891, w869) -> (→"Graph 2":T25)
    n979 = Build Array (concatenate)(w904, w903, w889, w867) -> (→"Graph 4":T25)
    n980 = Send Notification(notification="Stop Button", notifier=w829, error in (no error)=w828) -> (notifier out=w825:refnum<notifier>, error out=w826:errorcluster)
    "Cycle #" <- w837
  }
  n981 = while {
    tunnel: w3 -> [w2022]
    tunnel: w2 -> [w2021]
    stop <- w2023 stop-if-true
    n982 = Wait (ms)(milliseconds to wait=u32 214) -> ()  [unwired: 1 out]
    n983 = case shown="True" "RECORD GRAPH" {
      frame False {
      }
      frame True {
        n984 = stacked-sequence {
          frame #0 {
            n985 = Get Date/Time In Seconds() -> (seconds since 1Jan1904=w2044:timestamp)
            n986 = local read "Base Path"() -> (w2029:path)
            n987 = local read "RUN Identifier"() -> (w2045:string)
            n988 = call "LV_UNIXTIME.vi"("current time"=w2044) -> ("date/time string"=w2046:string)  [unwired: 9 in, 1 out]
            n989 = control-ref of="Graph CHF"() -> (w2035:refnum<vi>)
            n990 = Concatenate Strings(w2045, "_CHF" ("string"), w2046, "_" ("string"), "CHF Graph Comment") -> (w2031:string)
            n991 = Concatenate Strings(w2031, ".png" ("string")) -> (w2030:string)
            n992 = Concatenate Strings(w2031, ".csv" ("string")) -> (w2033:string)
            "CHF file name" <- w2033
            n993 = Build Path(base path=w2029, name or relative path=w2033) -> (appended path=w2040:path)
            n994 = invoke class="XYGraph (strict)" method="Get Image"(reference=w2035) -> ("image data"=w2027:T23)  [unwired: 5 in, 5 out]
            n995 = local read "ƒ¢T_array"() -> (w2037:dbl[])
            n996 = local read "Q_array"() -> (w2036:dbl[])
            n997 = Build Path(base path=w2029, name or relative path=w2030) -> (appended path=w2028:path)
            n998 = Open/Create/Replace File(file path (use dialog)=w2040, operation (0:open)=T24."open or create") -> (refnum out=w2038:refnum<file>)  [unwired: 4 in, 2 out]